vi "optimize crop parameters-3 (SubVI).vi"(6 "ref image in":u16[][](array[numeric])=array300x57[17100 elements], 7 "fit results":bool=TRUE, 8 "init values":dbl[][][](array[numeric]), 9 "use external int values":bool, 10 "config in":T4={"xy cut pos correct"=[[0.0], [0.0], [0.0], [0.0], [0.0], [0.0], [0.0], [0.0], [0.0], [0.0], [0.0], [0.0], [0.0], [0.0], [0.0], [0.0], [0.0], [0.0], [0.0], [0.0], [0.0], [0.0], [0.0], [0.0], [0.0], [0.0], [0.0], [0.0], [0.0], [0.0], [0.0], [0.0], [0.0], [0.0], [0.0], [0.0], [0.0], [0.0], [0.0], [0.0]], "3D reconst config"={"xyz pos"=[0, 69, 24], "color 4"={"color array"=[0, 8388736, 16711680, 16776960, 16776960, 16711680, 16448250, 16448250], "num of colors"=4, "max"=7000.900000000023, "min"=100.0}, "autogain"=TRUE, "zoom"=1.0, "slice(T)/stack(F)"=FALSE, "xy cut mag"=0.999999999999986, "xy cut ofst"=0.0, "z/xy comp"=0.9999999999999996, "y shift comp"=-7.0, "max plot"=TRUE, "oblique angle [deg]"=0.0, "voxel size z [um]"=0.36775838497734437, "voxel size xy[um]"=0.20475, "reverse v"=FALSE, "reverse h"=TRUE, "3D reconstruction"=TRUE, "reverse z"=FALSE}, "xy cut pos"=[[0.0], [54.34536278984456], [110.7007419058657], [167.1825518682615], [222.80744164966734], [279.667373495206], [337.55045867160084], [394.00066092240456], [449.7285684304855], [506.4608987736647], [563.3091240593538], [619.1119535504733], [675.221494909653], [732.8446944573865], [789.812326653542], [845.898454893022], [902.613225396426], [960.3441252947761], [1016.341283679399], [1071.7472607916166], [1127.5653088105405], [1184.377243760696], [1240.3662075534241], [1296.3844377457767], [1353.119109400925], [1408.8200918213527], [1464.8184208619614], [1521.6959125472738], [1579.4607614691888], [1635.079797970669], [1691.0593965155172], [1748.3068154920788], [1805.199525705196], [1861.439009878706], [1917.7054191398715], [1974.9902991079516], [2031.335142320107], [2087.3943454719315], [2144.892284829274], [2201.6960251875375]], "AOD scan speed ratio"=10.0, "Nx"=56.85, "stack method"=enum."0pad to x", "y shift"=-3}, 11 "image in":u16[][][](array[numeric])=array1x300x2304[691200 elements]) -> (0 "opt param for feedback":dbl[][][](array[numeric])=[[[0.39047108985224355, 1.3701514145414102, -2.528506798772906, -0.14203827683511228, 5186038.086192495]], [[0.5290682113405143, 1.6501694868561811, -2.655816972530653, -0.1554672078248204, 6667073.766870199]], [[0.41314522689268984, 2.088686528657111, -2.792705091791418, -0.12569963497559422, 6491844.329115606]], [[0.8227560588149236, 1.8428855088240716, -2.628942466676763, -0.08668976787454216, 5631903.835843649]], [[0.32325175994989747, 1.2513074134525095, -1.6297905856914976, -0.1614369028609812, 7505225.271223895]], [[-0.003655911531680436, 0.19950104929288875, -1.7514530723749357, -0.08884972633189654, 5034310.712258729]], [[0.34354411314901734, 1.2590913467770888, -2.7890670826012935, -0.10927959716588379, 6468144.578476399]], [[-0.0310203421500183, 0.7829252064146169, -2.2702759490200592, -0.09899784044930304, 4653169.175374532]], [[0.14511870715681918, 0.24470450605468053, -1.7093878850525326, -0.06709896777407671, 5134381.833655705]], [[-0.003971505084047196, 0.7523626416256568, -1.534678939554147, -0.09611567176314631, 4740038.50089103]], [[-0.02792801163393208, -0.3890095646502043, -2.2976472939935375, -0.09700731789796588, 5338166.755682839]], [[-0.6560035416703861, -0.4121475704316506, -1.8006560477706657, -0.08317774197600952, 4965586.880682849]], [[-0.07899279410231272, 0.5752260971778136, -0.6710344360087989, -0.06849372931756358, 4655084.0858172625]], [[-0.05083354360854886, 0.2532900218711269, -1.39597945278722, -0.07627262365560383, 5236824.424857916]], [[-0.04837211414479735, 0.3406051408186316, -0.7975973572536321, -0.08658047534428787, 4753028.594224306]], [[-0.4313850295473879, -0.6276284625697358, -0.7897096438499904, -0.072834398097467, 4874063.437715337]], [[-0.46049782115417903, -0.2341675376827123, -0.7412505694712552, -0.08633169971762658, 5141070.08632244]], [[0.08833028483609733, 0.8215796169595931, -0.01775522596758547, -0.06738233458537551, 4677016.607236656]], [[-0.6223872033178044, -0.9987743136212477, -1.0676478560072118, -0.03407086417350795, 5553505.071871417]], [[-0.017060112368393276, 1.0784317210282457, -0.2722875991586168, -0.0816359092925706, 4696857.4358025845]], [[0.0, 0.0, 0.0, 0.0, 0.0]], [[-0.23613314760922, 0.3409617993905103, 0.3289119936344964, -0.09632032650540112, 5128288.939512947]], [[-0.35196031039538767, 0.10630624968944505, 0.8300543336834989, -0.08524955580697285, 4993967.3927470865]], [[-0.029822860931065412, 0.5761693339828244, 0.009485866537335071, -0.072483002212926, 4951118.4930408215]], [[0.3466422521632596, 1.1972939848079962, 0.8529442246259615, -0.08204563144140758, 4738224.722203573]], [[-0.5161452276940326, -0.4062966847061925, 1.4794783929753714, -0.04368130498426906, 4589002.30593094]], [[-0.38498865045824193, 0.7296022962419677, 1.219223749125252, -0.08128900584448218, 5155405.171288024]], [[0.39664586657630685, 0.19347099987965855, 1.9179908940418189, -0.08728195443943998, 5146203.651410466]], [[-0.06294995676019306, 0.5468584220156103, 1.258683657908979, -0.07957290144422699, 4724989.578754336]], [[-0.5068124364570108, -0.08803959075677643, 2.2015231672130584, -0.07409643531910859, 4765076.553921852]], [[-0.007101178214248816, 0.10218423404460837, 2.4109047574004157, -0.06616032890532567, 4331638.820783317]], [[-0.41299002227983295, 1.1421701438972842, 1.8680971965858637, -0.10395219837168257, 5779592.647707423]], [[-0.04906443565345491, 0.2939222046041641, 1.9091893754914997, -0.04341744032696582, 4796031.169651782]], [[-0.06496644337617823, 0.5511641655160622, 1.91046003816149, -0.05321838499215621, 4379387.893441995]], [[-0.3555959703865873, 0.1452031874907217, 3.037388781526421, -0.052724460570182485, 4931796.160483034]], [[-0.4774462977628986, -0.44051726867204, 2.350105869256047, -0.0908046301186699, 5146929.721792191]], [[-0.45397018791592364, 0.3915383175697266, 3.3398737812628516, -0.07691847566668765, 4864469.550526747]], [[0.14328180351502526, 0.3855249139291015, 2.6047417917604205, -0.06972164986512942, 4334268.987205673]], [[-0.07403056676163042, 0.8482394818552436, 3.2115811981035, -0.09535149758334224, 4409611.6475773165]], [[-0.26001393141243034, 0.5649152359263228, 4.100365157728029, -0.09799498059142073, 5159717.129331669]]], 3 "optimized parameters":dbl[][][](array[numeric])=[[[0.6536916642864307, 9.691050019608873, -3.146642560188741, -0.1502911301649359]], [[0.5397363402674268, 65.0684934356392, -2.979252154665359, -0.13747551755601403]], [[0.4364891379835099, 120.61174935417779, -2.8118617491419773, -0.12770796069082646]], [[0.3433633747841549, 176.2986144777129, -2.644471343618595, -0.12005961729517042]], [[0.259784258948234, 232.1081618516672, -2.477080938095213, -0.11381811925822599]], [[0.18518888968401584, 288.0207408643976, -2.309690532571831, -0.10845694075667886]], [[0.11902625712916581, 344.01797724719563, -2.142300127048449, -0.1036067632845281]], [[0.06075724235074598, 400.08277307428693, -1.974909721525067, -0.0990288375885783]], [[0.009854617345215477, 456.19930676283155, -1.8075193160016851, -0.09459034250961632]], [[-0.03419695496157027, 512.353033072924, -1.6401289104783032, -0.09024174072927313]], [[-0.071900920714359, 568.5306831075931, -1.472738504954921, -0.0859961314225699]], [[-0.10374883512850164, 624.720264312802, -1.3053480994315392, -0.08191059981614907]], [[-0.1302203624899524, 680.9110604774485, -1.1379576939081573, -0.07806956365218976]], [[-0.15178327615526876, 737.0936317333643, -0.9705672883847751, -0.07457011655800833]], [[-0.16889345855161175, 793.2598145553159, -0.803176882861393, -0.07150936832134314]], [[-0.1819949011767451, 849.4027217610037, -0.6357864773380113, -0.06897378207132454]], [[-0.19151970459903644, 905.5167425110632, -0.46839607181462917, -0.06703050836512858]], [[-0.19788807845745615, 961.5975423090633, -0.30100566629124703, -0.06572071618031705]], [[-0.20150834146157814, 1017.6420630015082, -0.13361526076786534, -0.0650549208128599]], [[-0.20277692139158043, 1073.6485227778358, 0.033775144755516795, -0.06501030868084456]], [[-0.20207835509824212, 1129.6164161704187, 0.20116555027889893, -0.06553005903386944]], [[-0.1997852885029483, 1185.5465140545639, 0.3685559558022806, -0.06652466256812017]], [[-0.19625847659768425, 1241.440863648512, 0.5359463613256628, -0.06787523694713249]], [[-0.1918467834450428, 1297.3027885134397, 0.7033367668490449, -0.06943883922824079]], [[-0.1868871821782152, 1353.1368885534564, 0.8707271723724266, -0.07105577519470918]], [[-0.18170475500099958, 1408.9490400156064, 1.0381175778958087, -0.07255890559354494]], [[-0.17661269318779516, 1464.7463954898685, 1.2055079834191909, -0.07378494927900459]], [[-0.1719122970836069, 1520.537383909156, 1.372898388942573, -0.07458778326177828]], [[-0.16789297610403953, 1576.3317105493163, 1.5402887944659551, -0.07485373966385556]], [[-0.1648322487353049, 1632.1403570291309, 1.7076791999893364, -0.07451889957908975]], [[-0.16299574253421412, 1687.9755813103163, 1.8750696055127185, -0.07358838383942778]], [[-0.16263719412818567, 1743.850917697523, 2.0424600110361006, -0.07215764068684027]], [[-0.1639984492152391, 1799.781176838336, 2.2098504165594828, -0.07043573035093509]], [[-0.16730946256399637, 1855.7824457232746, 2.377240822082865, -0.06877060653223754]], [[-0.172788298013685, 1911.8720876857924, 2.544631227606247, -0.06767639479118515]], [[-0.18064112847413405, 1968.0687424022772, 2.712021633129629, -0.06786266784277828]], [[-0.1910622359257763, 2024.392325892052, 2.8794120386530104, -0.07026571775693569]], [[-0.2042340114196488, 2080.864030517373, 3.0468024441763926, -0.07608182506452543]], [[-0.22032695507739053, 2137.506324983432, 3.2141928496997747, -0.08680252476907313]], [[-0.23949967609124334, 2194.342954338354, 3.381583255223157, -0.10425186926418739]]])   [LabVIEW 2024]
uses:
  <vilib>/Analysis/6fits.llb/General Linear Fit Algorithm.ctl
  <vilib>/Analysis/6fits.llb/Curve Fitting Criteria.ctl
  <vilib>/Analysis/1siggen.llb/Ramp Pattern by Samples.vi
  Global variables/global for picoscope.vi
  <vilib>/gmath/NumericalOptimization/Conjugate Gradient.vi
  <vilib>/gmath/NumericalOptimization/Downhill Simplex.vi
  <vilib>/gmath/NI_Gmath.lvlib
  <vilib>/Analysis/NI_AALBase.lvlib
  <vilib>/Analysis/NI_AALPro.lvlib
panel:
  out "y correct":dbl[](array[numeric])
  out "intensity correct fit":dbl[][](graph)=[[-0.008252853329823617, 0.01799169026880637, -0.00200832571523224, -0.03336984942062826, 0.047618783602755205, -0.019607214424782318, 0.005672833881355685, -3.099713927526282e-05, -0.0274913747355396, 0.005873931033873181, 0.011011186475395979, 0.001267142159860457, -0.00957583433462618, 0.001702507097595507, 0.01507110702294473, 0.0038606160261424605, 0.019301191352498, 0.0016616184050584626, -0.030984056639351956, 0.016625600611726035, -0.06553005903386944, 0.029795663937280947, 0.017374318859840365, 0.0030441629846852114, 0.010989856246698404, -0.028877600609275883, 0.00750405656547759, 0.012694171177661695, 0.004719161780371434, -0.000422464259981159, -0.0074280549341021185, 0.031794557684842295, -0.02701829002396927, -0.015552221540081332, -0.01495193422100266, 0.022941962275891625, 0.0066527579097519635, -0.006360175199396009, 0.008548972814269112, -0.006256888672766664]]
  out "y correct fit":dbl[][](graph)=[[-0.6181357614158349, -0.3234351821347059, -0.01915665735055949, -0.015528876941832248, -0.8472903524037154, -0.5582374601968951, 0.6467669555528444, 0.2953662274949922, -0.09813143094915255, -0.10544997092415631, 0.8249087890386164, 0.4953079483391265, -0.4669232578993584, 0.4254121644024449, -0.005579525607760871, 0.15392316651197913, 0.27285449765662606, -0.28325044032366153, 0.9340325952393465, 0.3060627439141336, 0.20116555027889893, 0.03964396216778421, -0.29410797235783614, 0.6938509003117098, 0.01778294774646505, -0.4413608150795627, -0.013715765706061145, -0.5450925050992459, 0.28160513655697605, -0.49384396722372204, -0.5358351518876971, 0.17436281445023694, 0.3006610410679831, 0.4667807839213749, -0.49275755392017384, 0.3619157638735824, -0.4604617426098412, 0.44206065241597203, 0.0026116515962746334, -0.7187819025048721]]
  out "r correct fit":dbl[][](graph)=[[0.2632205744341871, 0.01066812892691249, 0.02334391109082007, -0.47939268403076873, -0.06346750100166348, 0.18884480121569627, -0.22451785601985152, 0.09177758450076427, -0.1352640898116037, -0.030225449877523073, -0.04397290908042692, 0.5522547065418845, -0.05122756838763967, -0.1009497325467199, -0.1205213444068144, 0.24939012837064278, 0.2689781165551426, -0.2862183632935535, 0.42087886185622625, -0.18571680902318716, -0.20207835509824212, 0.036347859106271696, 0.15570183379770342, -0.1620239225139774, -0.5335294343414748, 0.334440472693033, 0.20837595727044678, -0.5685581636599137, -0.10494301934384646, 0.3419801877217059, -0.1558945643199653, 0.2503528281516473, -0.11493401356178418, -0.10234301918781814, 0.1828076723729023, 0.29680516928876455, 0.2629079519901473, -0.3475158149346741, -0.1462963883157601, 0.020514255321187003]]
  out "x cut pos fit":dbl[][](graph)=[[0.05958342353034496, 0.3696472414168426, -0.5619591246160951, -0.507951857113909, -0.017269990121718592, 1.1759828176153064, -0.5767823185710199, -0.6787897339829101, 0.46230636415401705, -0.4421715948110432, 0.704871654653175, 1.0956096058057483, 0.08464138025601642, 0.2628733892471473, -0.6385644162365907, 0.6061678936717954, -0.22042479817071126, -1.4538074471773825, -0.10131294393795542, -1.3327500488101123, 0.5811761866887082, -0.25952303329358983, 0.5225790325855542, 0.27997021796568333, -1.2632396330939173, 1.5644171407125214, 0.3021165107622892, -0.17226765343639272, 0.22220656651415993, 0.9923966661572194, 0.7340449659257047, -0.6067568190055681, -0.3854211309949278, -0.34487591421111574, -0.3506291171152043, 0.27174445488094534, -0.9228543205397273, -0.358506167194264, 0.28250261545827016, 0.6210199346419358]]
  out "x cut correct 3":dbl[](graph)=[1.3701514145414102, 1.6501694868561811, 2.088686528657111, 1.8428855088240716, 1.2513074134525095, 0.19950104929288875, 1.2590913467770888, 0.7829252064146169, 0.24470450605468053, 0.7523626416256568, -0.3890095646502043, -0.4121475704316506, 0.5752260971778136, 0.2532900218711269, 0.3406051408186316, -0.6276284625697358, -0.2341675376827123, 0.8215796169595931, -0.9987743136212477, 1.0784317210282457, 0.0, 0.3409617993905103, 0.10630624968944505, 0.5761693339828244, 1.1972939848079962, -0.4062966847061925, 0.7296022962419677, 0.19347099987965855, 0.5468584220156103, -0.08803959075677643, 0.10218423404460837, 1.1421701438972842, 0.2939222046041641, 0.5511641655160622, 0.1452031874907217, -0.44051726867204, 0.3915383175697266, 0.3855249139291015, 0.8482394818552436, 0.5649152359263228]
  out "x cut correct 2":dbl[](graph)=[-0.8029671311863609, -1.22048533842898, -0.20099096700753716, -2.396117725234003, -0.5704273524019985, 0.2214525690458135, -0.6696516702608777, 0.9702091819145723, -0.6014491907781662, 0.7762106145991239, -0.22050026893236452, 4.118267322604225, 1.0567908915209814, 0.5614239918423856, 0.6336730889351082, 2.205079255222368, 2.8091033079627183, 0.30079806451595614, 3.266476398749979, 1.1811428479118296, 0.0, 1.827987916571229, 2.3779756021428033, 0.756180187298116, -0.7477150646922253, 3.0470615566129515, 3.2322309224736365, -2.0114867259898572, 0.9293740307831726, 3.295832744570641, 0.1448519014721809, 3.843210849841621, 0.5912262293633566, 0.9460942665828354, 2.4421349452744177, 2.7265847440253017, 3.387362410336551, -0.45021659697024496, 1.2990983499316635, 2.2105778664701514]
  out "size(s)":i32[](array[numeric])=[40, 1]
  out "loss function":dbl[](graph)=[5186038.086192495, 6667073.766870199, 6491844.329115606, 5631903.835843649, 7505225.271223895, 5034310.712258729, 6468144.578476399, 4653169.175374532, 5134381.833655705, 4740038.50089103, 5338166.755682839, 4965586.880682849, 4655084.0858172625, 5236824.424857916, 4753028.594224306, 4874063.437715337, 5141070.08632244, 4677016.607236656, 5553505.071871417, 4696857.4358025845, 0.0, 5128288.939512947, 4993967.3927470865, 4951118.4930408215, 4738224.722203573, 4589002.30593094, 5155405.171288024, 5146203.651410466, 4724989.578754336, 4765076.553921852, 4331638.820783317, 5779592.647707423, 4796031.169651782, 4379387.893441995, 4931796.160483034, 5146929.721792191, 4864469.550526747, 4334268.987205673, 4409611.6475773165, 5159717.129331669]
  out "intensity correct":dbl[][](graph)=[[-0.14203827683511228, -0.1554672078248204, -0.12569963497559422, -0.08668976787454216, -0.1614369028609812, -0.08884972633189654, -0.10927959716588379, -0.09899784044930304, -0.06709896777407671, -0.09611567176314631, -0.09700731789796588, -0.08317774197600952, -0.06849372931756358, -0.07627262365560383, -0.08658047534428787, -0.072834398097467, -0.08633169971762658, -0.06738233458537551, -0.03407086417350795, -0.0816359092925706, 0.0, -0.09632032650540112, -0.08524955580697285, -0.072483002212926, -0.08204563144140758, -0.04368130498426906, -0.08128900584448218, -0.08728195443943998, -0.07957290144422699, -0.07409643531910859, -0.06616032890532567, -0.10395219837168257, -0.04341744032696582, -0.05321838499215621, -0.052724460570182485, -0.0908046301186699, -0.07691847566668765, -0.06972164986512942, -0.09535149758334224, -0.09799498059142073], [-0.1502911301649359, -0.13747551755601403, -0.12770796069082646, -0.12005961729517042, -0.11381811925822599, -0.10845694075667886, -0.1036067632845281, -0.0990288375885783, -0.09459034250961632, -0.09024174072927313, -0.0859961314225699, -0.08191059981614907, -0.07806956365218976, -0.07457011655800833, -0.07150936832134314, -0.06897378207132454, -0.06703050836512858, -0.06572071618031705, -0.0650549208128599, -0.06501030868084456, -0.06553005903386944, -0.06652466256812017, -0.06787523694713249, -0.06943883922824079, -0.07105577519470918, -0.07255890559354494, -0.07378494927900459, -0.07458778326177828, -0.07485373966385556, -0.07451889957908975, -0.07358838383942778, -0.07215764068684027, -0.07043573035093509, -0.06877060653223754, -0.06767639479118515, -0.06786266784277828, -0.07026571775693569, -0.07608182506452543, -0.08680252476907313, -0.10425186926418739]]
  out "y correct":dbl[][](graph)=[[-2.528506798772906, -2.655816972530653, -2.792705091791418, -2.628942466676763, -1.6297905856914976, -1.7514530723749357, -2.7890670826012935, -2.2702759490200592, -1.7093878850525326, -1.534678939554147, -2.2976472939935375, -1.8006560477706657, -0.6710344360087989, -1.39597945278722, -0.7975973572536321, -0.7897096438499904, -0.7412505694712552, -0.01775522596758547, -1.0676478560072118, -0.2722875991586168, 0.0, 0.3289119936344964, 0.8300543336834989, 0.009485866537335071, 0.8529442246259615, 1.4794783929753714, 1.219223749125252, 1.9179908940418189, 1.258683657908979, 2.2015231672130584, 2.4109047574004157, 1.8680971965858637, 1.9091893754914997, 1.91046003816149, 3.037388781526421, 2.350105869256047, 3.3398737812628516, 2.6047417917604205, 3.2115811981035, 4.100365157728029], [-3.146642560188741, -2.979252154665359, -2.8118617491419773, -2.644471343618595, -2.477080938095213, -2.309690532571831, -2.142300127048449, -1.974909721525067, -1.8075193160016851, -1.6401289104783032, -1.472738504954921, -1.3053480994315392, -1.1379576939081573, -0.9705672883847751, -0.803176882861393, -0.6357864773380113, -0.46839607181462917, -0.30100566629124703, -0.13361526076786534, 0.033775144755516795, 0.20116555027889893, 0.3685559558022806, 0.5359463613256628, 0.7033367668490449, 0.8707271723724266, 1.0381175778958087, 1.2055079834191909, 1.372898388942573, 1.5402887944659551, 1.7076791999893364, 1.8750696055127185, 2.0424600110361006, 2.2098504165594828, 2.377240822082865, 2.544631227606247, 2.712021633129629, 2.8794120386530104, 3.0468024441763926, 3.2141928496997747, 3.381583255223157]]
  out "x cut pos":dbl[][](graph)=[[9.631466596078528, 64.69884619422236, 121.17370847879388, 176.8065663348268, 232.12543184178892, 286.8447580467823, 344.59475956576665, 400.76156280826984, 455.73700039867754, 512.795204667735, 567.8258114529399, 623.6246547069962, 680.8264190971925, 736.8307583441172, 793.8983789715525, 848.7965538673319, 905.7371673092339, 963.0513497562407, 1017.7433759454461, 1074.9812728266459, 1129.03523998373, 1185.8060370878575, 1240.9182846159265, 1297.022818295474, 1354.4001281865503, 1407.384622874894, 1464.4442789791062, 1520.7096515625924, 1576.1095039828022, 1631.1479603629737, 1687.2415363443906, 1744.4576745165286, 1800.166597969331, 1856.1273216374857, 1912.2227168029076, 1967.7969979473962, 2025.3151802125917, 2081.2225366845673, 2137.2238223679738, 2193.721934403712], [9.691050019608873, 65.0684934356392, 120.61174935417779, 176.2986144777129, 232.1081618516672, 288.0207408643976, 344.01797724719563, 400.08277307428693, 456.19930676283155, 512.353033072924, 568.5306831075931, 624.720264312802, 680.9110604774485, 737.0936317333643, 793.2598145553159, 849.4027217610037, 905.5167425110632, 961.5975423090633, 1017.6420630015082, 1073.6485227778358, 1129.6164161704187, 1185.5465140545639, 1241.440863648512, 1297.3027885134397, 1353.1368885534564, 1408.9490400156064, 1464.7463954898685, 1520.537383909156, 1576.3317105493163, 1632.1403570291309, 1687.9755813103163, 1743.850917697523, 1799.781176838336, 1855.7824457232746, 1911.8720876857924, 1968.0687424022772, 2024.392325892052, 2080.864030517373, 2137.506324983432, 2194.342954338354]]
  out "r correct":dbl[][](graph)=[[0.39047108985224355, 0.5290682113405143, 0.41314522689268984, 0.8227560588149236, 0.32325175994989747, -0.003655911531680436, 0.34354411314901734, -0.0310203421500183, 0.14511870715681918, -0.003971505084047196, -0.02792801163393208, -0.6560035416703861, -0.07899279410231272, -0.05083354360854886, -0.04837211414479735, -0.4313850295473879, -0.46049782115417903, 0.08833028483609733, -0.6223872033178044, -0.017060112368393276, 0.0, -0.23613314760922, -0.35196031039538767, -0.029822860931065412, 0.3466422521632596, -0.5161452276940326, -0.38498865045824193, 0.39664586657630685, -0.06294995676019306, -0.5068124364570108, -0.007101178214248816, -0.41299002227983295, -0.04906443565345491, -0.06496644337617823, -0.3555959703865873, -0.4774462977628986, -0.45397018791592364, 0.14328180351502526, -0.07403056676163042, -0.26001393141243034], [0.6536916642864307, 0.5397363402674268, 0.4364891379835099, 0.3433633747841549, 0.259784258948234, 0.18518888968401584, 0.11902625712916581, 0.06075724235074598, 0.009854617345215477, -0.03419695496157027, -0.071900920714359, -0.10374883512850164, -0.1302203624899524, -0.15178327615526876, -0.16889345855161175, -0.1819949011767451, -0.19151970459903644, -0.19788807845745615, -0.20150834146157814, -0.20277692139158043, -0.20207835509824212, -0.1997852885029483, -0.19625847659768425, -0.1918467834450428, -0.1868871821782152, -0.18170475500099958, -0.17661269318779516, -0.1719122970836069, -0.16789297610403953, -0.1648322487353049, -0.16299574253421412, -0.16263719412818567, -0.1639984492152391, -0.16730946256399637, -0.172788298013685, -0.18064112847413405, -0.1910622359257763, -0.2042340114196488, -0.22032695507739053, -0.23949967609124334]]
  out "slice":i32=39
  out "page":i32
  out "Numeric":i32=9
  out "Waveform Graph 3":dbl[](graph)=[0.0, 0.0, 7.072244388269059e-25, 0.0, 0.0, 1251222.7679371487, 0.0, 0.0, 0.0, 1886418.1063101203]
  out "x-y":dbl=6.488273299997672
  out "sum 2":dbl
  out "difference from ref img":dbl[][](graph)
  out "error out":errorcluster
  in  "Conjugate gradient settings":T1
  in  "Stopping criteria":T2={"function tolerance"=1000.0, "parameter tolerance"=0.1, "max iterations"=1000, "max function calls"=1000, "gradient tolerance"=-1.0, "max time (sec)"=-1.0}
  in  "Optimization Method":T3(ring)=enum."Downhill Simplex"
  out "Number of function evaluations":i32=89
  out "Minimum":dbl[](array[numeric])
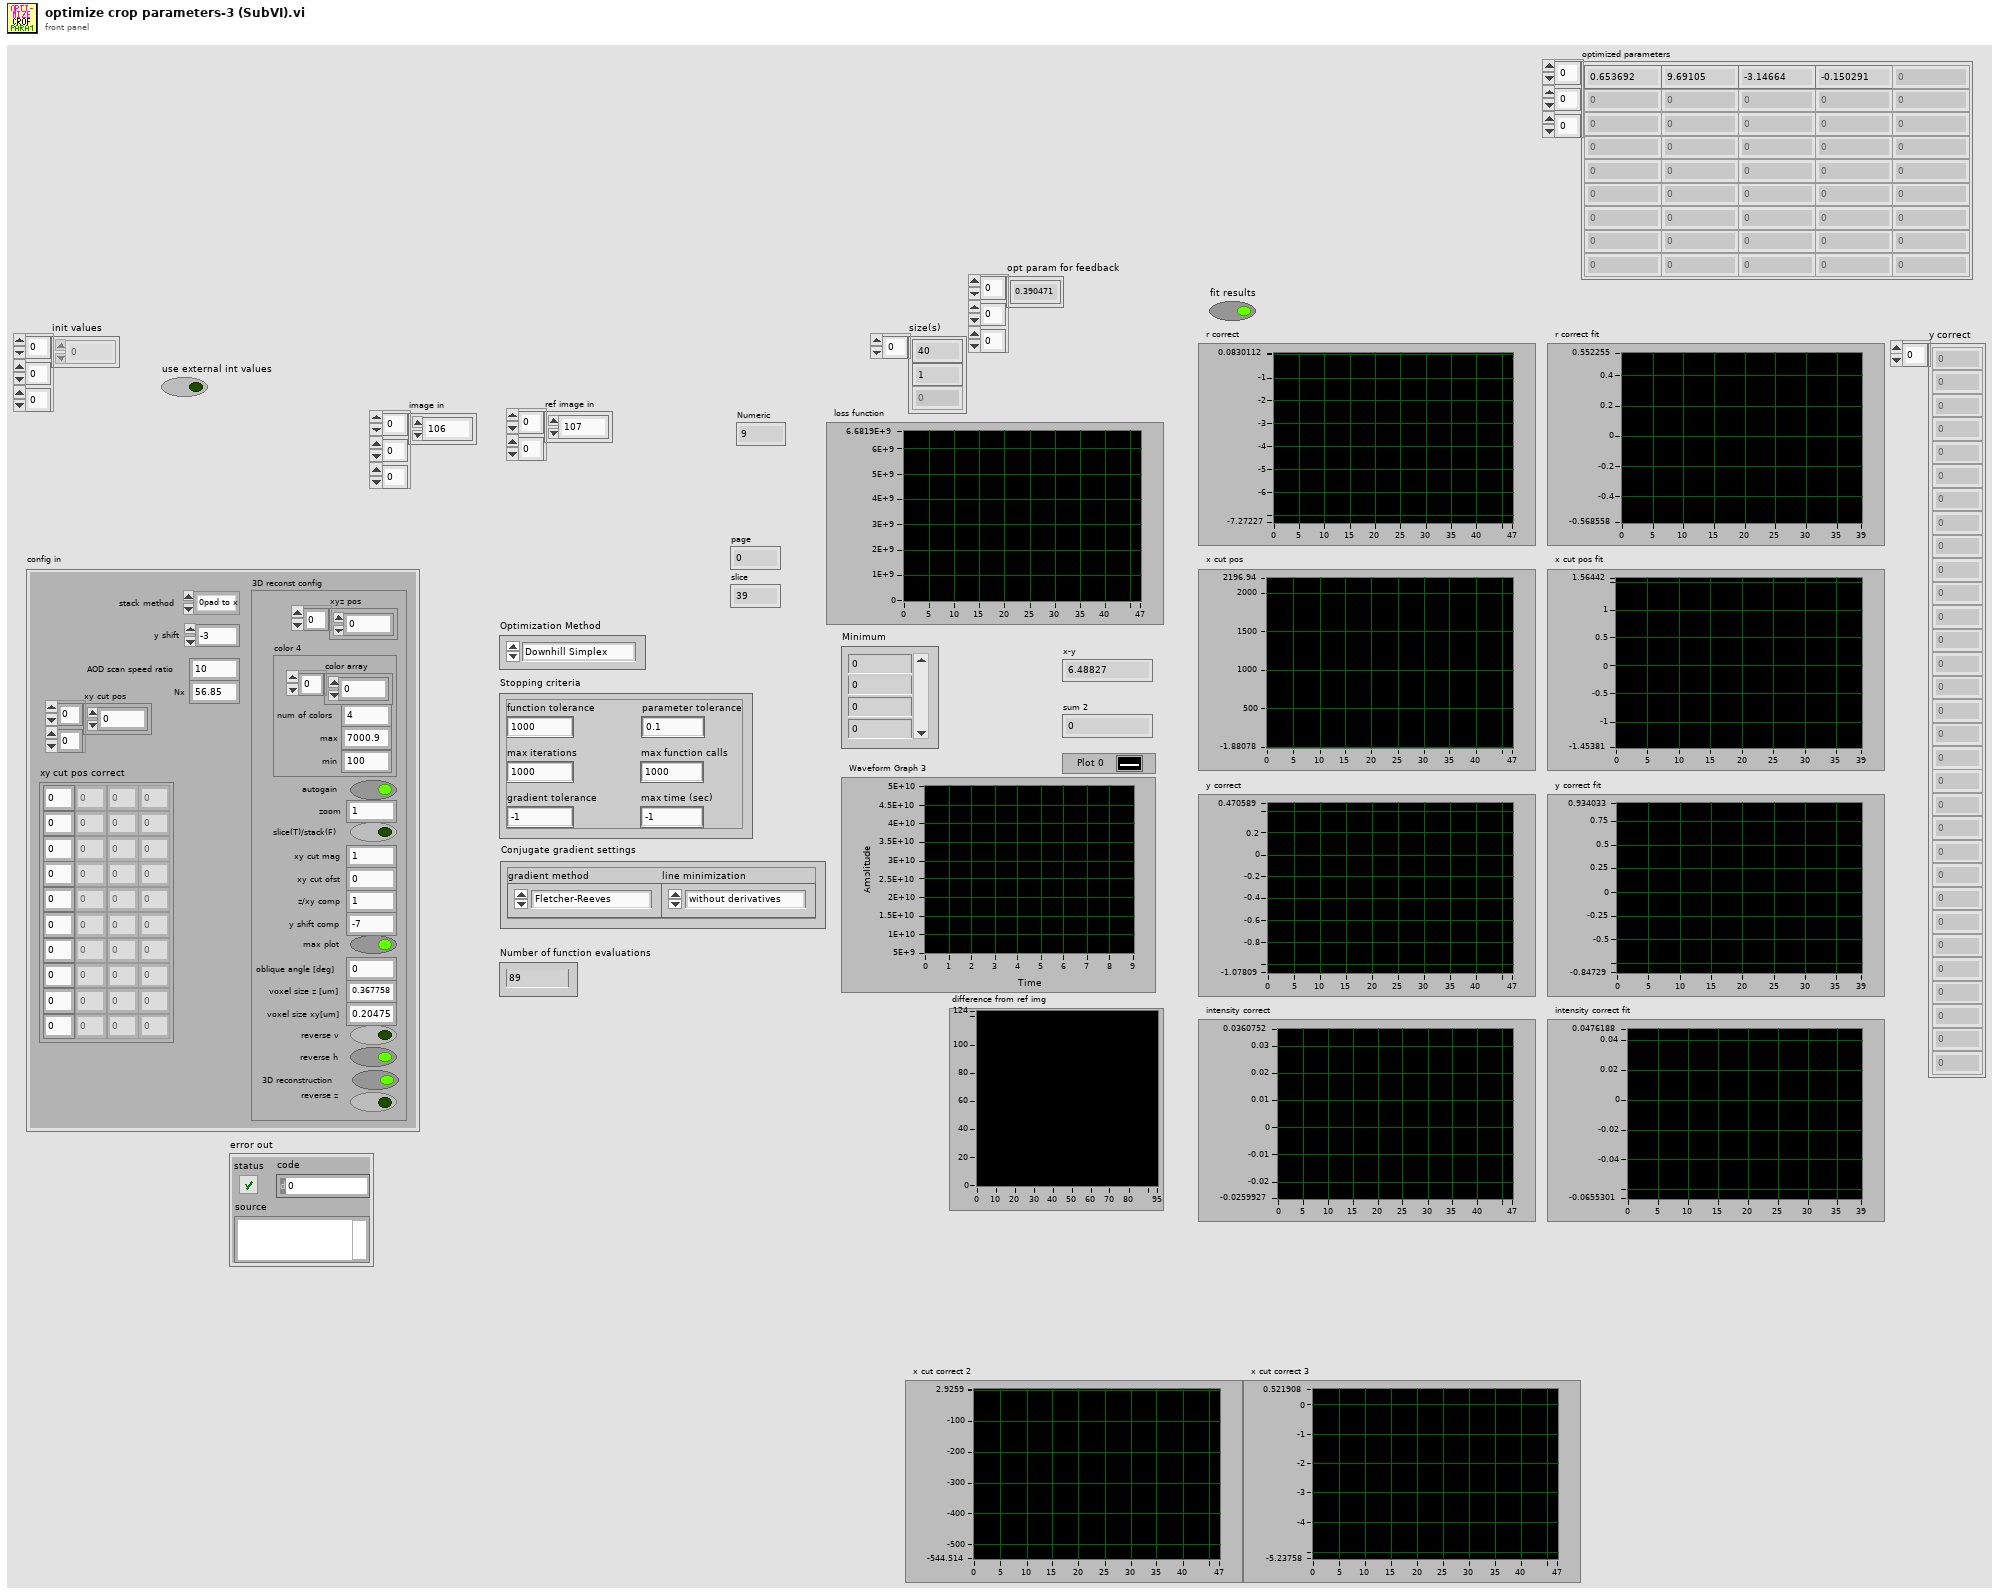
[diagram p1: front panel]
types:
  T1 = cluster{"gradient method":enum16{"Fletcher-Reeves", "Polak-Ribiere"}, "line minimization":enum16{"without derivatives", "with derivatives"}}
  T2 = cluster{"function tolerance":dbl, "parameter tolerance":dbl, "max iterations":i32, "max function calls":i32, "gradient tolerance":dbl, "max time (sec)":dbl}
  T3 = enum16{"Quasi-newton", "Conjugate Gradient", "Downhill Simplex"}
  T4 = cluster{"xy cut pos correct":dbl[][], "3D reconst config":cluster{"xyz pos":u16[], "color 4":cluster{"color array":u32[], "num of colors":i32, "max":dbl, "min":dbl}, "autogain":bool, "zoom":dbl, "slice(T)/stack(F)":bool, "xy cut mag":dbl, "xy cut ofst":dbl, "z/xy comp":dbl, "y shift comp":dbl, "max plot":bool, "oblique angle [deg]":dbl, "voxel size z [um]":dbl, "voxel size xy[um]":dbl, "reverse v":bool, "reverse h":bool, "3D reconstruction":bool, "reverse z":bool}, "xy cut pos":dbl[][], "AOD scan speed ratio":dbl, "Nx":dbl, "stack method":enum16{"0pad to z", "0pad to x", "0pad to x and rot"}, "y shift":i32}
  T5 = cluster{"xyz pos":u16[], "color 4":cluster{"color array":u32[], "num of colors":i32, "max":dbl, "min":dbl}, "autogain":bool, "zoom":dbl, "slice(T)/stack(F)":bool, "xy cut mag":dbl, "xy cut ofst":dbl, "z/xy comp":dbl, "y shift comp":dbl, "max plot":bool, "oblique angle [deg]":dbl, "voxel size z [um]":dbl, "voxel size xy[um]":dbl, "reverse v":bool, "reverse h":bool, "3D reconstruction":bool, "reverse z":bool}
  T6 = cluster{"GT":dbl[][], "frame input":u16[][], "cut pos init":dbl, "Nx":dbl, "r init":dbl}
  T7 = typedef "NI_AALPro.lvlib/General Linear Fit Algorithm.ctl" = u16
  T8 = typedef "NI_AALPro.lvlib/Curve Fitting Criteria.ctl" = u16
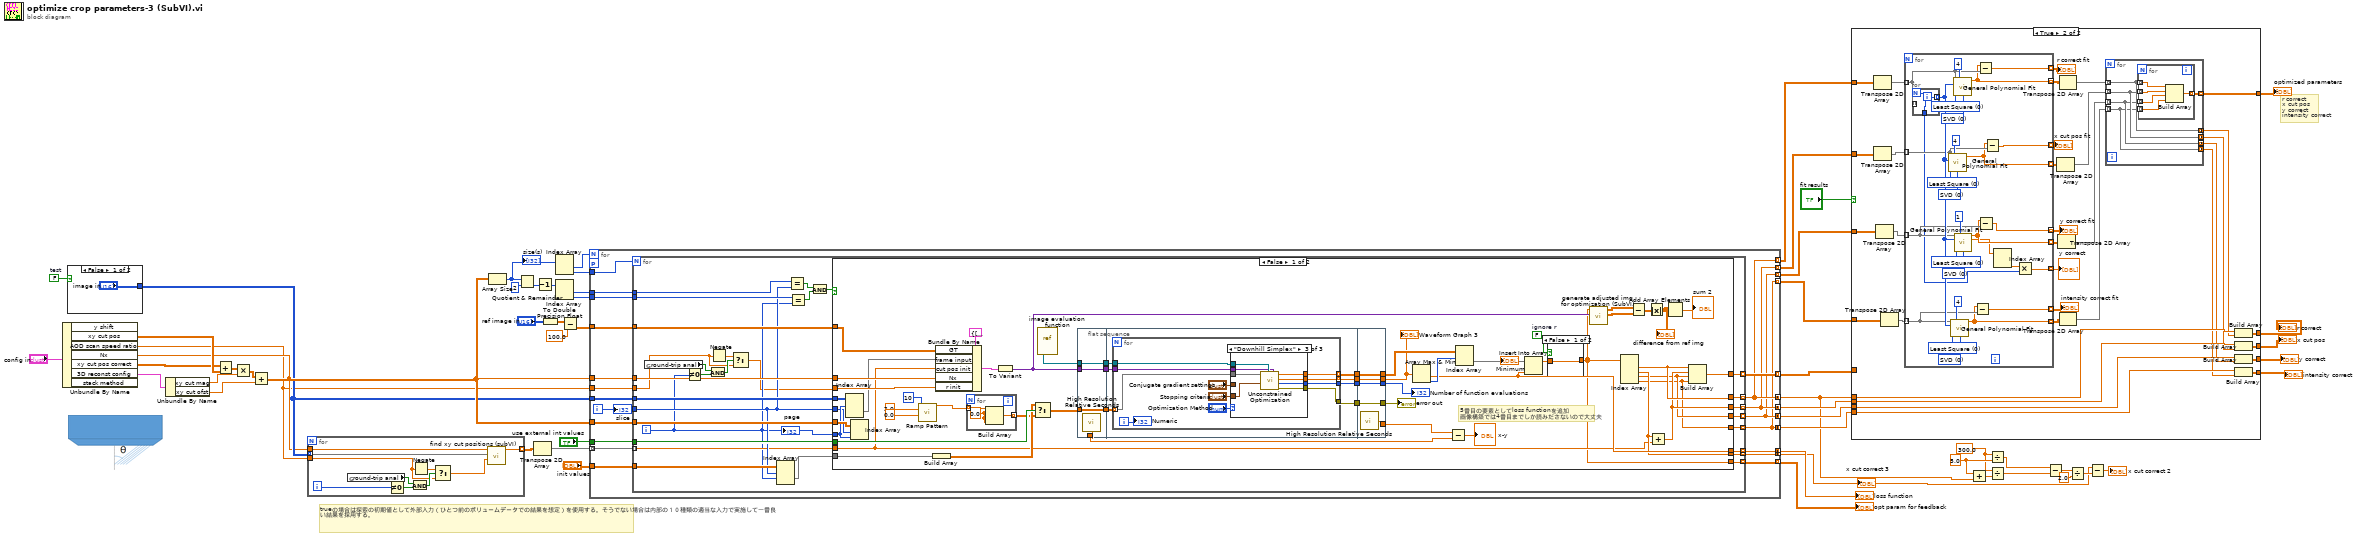
[diagram p0: block diagram]
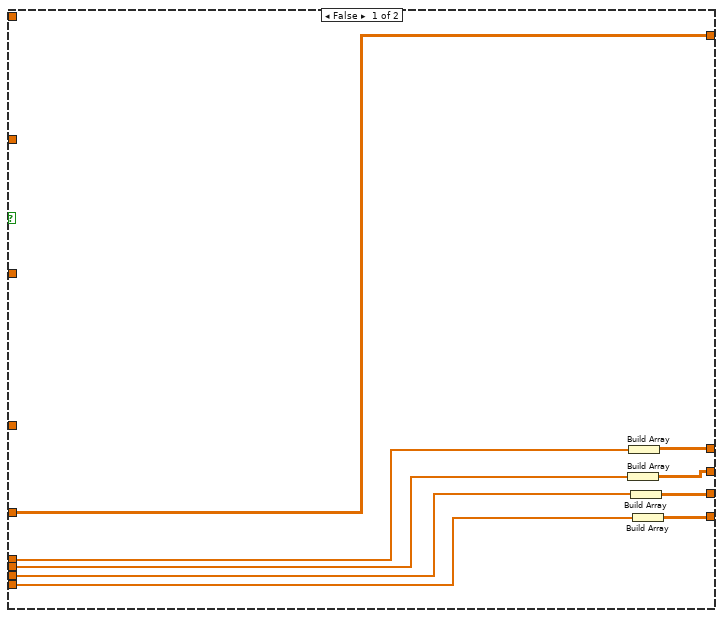
[diagram p2: hidden frame]
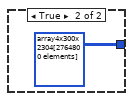
[diagram p3: hidden frame]
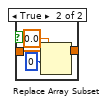
[diagram p4: hidden frame]
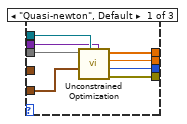
[diagram p5: hidden frame]
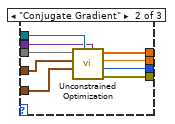
[diagram p6: hidden frame]
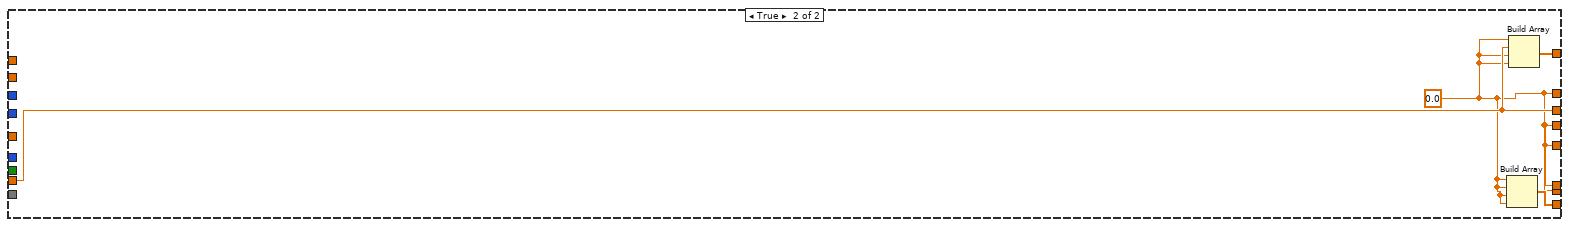
[diagram p7: hidden frame]
diagram:
  w28 = 5.0 ("y")
  w27 = 300.0 ("x")
  w37 = FALSE  # test
  # "r correct\nx cut pos\ny correct\nintensity correct"
  # "trueの場合は探索の初期値として外部入力（ひとつ前のボリュームデータでの結果を想定）を使用する。そうでない場合は内部の１０種類の適当な入力で実施して一番良い結果を採用する。"
  n1 = Unbundle By Name("config in") -> ("xy cut pos"=w55:dbl[][], "AOD scan speed ratio"=w33:dbl, "Nx"=w34:dbl, "xy cut pos correct"=w54:dbl[][], "3D reconst config"=w53:T5)  [unwired: 2 out]
  n2 = case shown="False" w37 {
    tunnel: ["image in" u16[][][] array4x300x2304[2764800 elements] ("Array out")] -> w35
    frame False {
    }
    frame True {
    }
  }
  n3 = Unbundle By Name(w53) -> ("xy cut mag"=w51:dbl, "xy cut ofst"=w49:dbl)
  n4 = Add(x=w54, y=w55) -> (x+y=w52:dbl[][])
  n5 = Multiply(x=w52, y=w51) -> (x*y=w50:dbl[][])
  n6 = Add(x=w50, y=w49) -> (x+y=w45:dbl[][])
  n7 = for {
    tunnel: w35 -> [w68] mode=indexing
    tunnel: w34 -> [w61]
    tunnel: w33 -> [w60]
    tunnel: [w67] -> w32 mode=indexing
    i -> [w63]
    n8 = global read "global for picoscope.vi" "round-trip anal"() -> (w64:bool)
    n9 = Not Equal To 0?(x=w63) -> (x != 0?=w62:bool)
    n10 = And(x=w64, y=w62) -> (x .and. y?=w65:bool)
    n11 = Negate(x=w60) -> (-x=w66:dbl)
    n12 = Select(t=w66, s=w65, f=w60) -> (s? t:f=w59:dbl)
    n13 = call "find xy cut positions (subVI).vi"("r"=w59, "input frame"=w68, "Nx"=w61) -> ("xy cut positions"=w67:dbl[])  [unwired: 7 in, 1 out]
  }
  n14 = Array Size(array=w45) -> (size(s)=w41:i32[])
  "size(s)" <- w41
  n15 = Quotient & Remainder(x=w41, y=2) -> (floor(x/y)=w43:i32[])  [unwired: 1 out]
  n16 = Transpose 2D Array(2D array=w32) -> (transposed array=w29:dbl[][])
  n17 = Decrement(x=w43) -> (x-1=w42:i32[])
  n18 = To Double Precision Float(number="ref image in") -> (double precision float=w48:dbl[][])
  n19 = Index Array(array=w41) -> (element #1=w17:i32, element #2=w16:i32)  [unwired: 2 in]
  n20 = Index Array(array=w42) -> (element #1=w39:i32, element #2=w38:i32)  [unwired: 2 in]
  n21 = Subtract(x=w48, y=100.0) -> (x-y=w46:dbl[][])
  n22 = for {
    N: w17 -> [_]
    tunnel: w35 -> [w88]
    tunnel: w34 -> [w87]
    tunnel: w33 -> [w86]
    tunnel: w46 -> [w85]
    tunnel: w45 -> [w84]
    tunnel: [w82] -> w10 mode=indexing
    tunnel: [w72] -> w1 mode=concatenating
    tunnel: [w81] -> w19 mode=concatenating
    tunnel: [w70] -> w7 mode=concatenating
    tunnel: [w69] -> w6 mode=concatenating
    tunnel: w16 -> [w78]
    tunnel: [w80] -> w40 mode=concatenating
    tunnel: w39 -> [w79]
    tunnel: w38 -> [w77]
    tunnel: "use external int values" -> [w76]
    tunnel: "init values" -> [w75]
    tunnel: w29 -> [w74] mode=indexing
    tunnel: [w71] -> w8 mode=concatenating
    tunnel: [w73] -> w18 mode=indexing
    tunnel: [w72] -> w15 mode=indexing
    tunnel: [w71] -> w14 mode=indexing
    tunnel: [w70] -> w13 mode=indexing
    tunnel: [w69] -> w12 mode=indexing
    workers-P: _ -> [_]
    i -> [w83]
    n23 = for {
      N: w78 -> [_]
      tunnel: w88 -> [w117]
      tunnel: w87 -> [w116]
      tunnel: w86 -> [w90]
      tunnel: w85 -> [w115]
      tunnel: w84 -> [w114]
      tunnel: w83 -> [w100]
      tunnel: [w113] -> w82 mode=indexing
      tunnel: [w112] -> w72 mode=indexing
      tunnel: [w111] -> w81 mode=indexing
      tunnel: [w110] -> w70 mode=indexing
      tunnel: [w109] -> w69 mode=indexing
      tunnel: [w108] -> w80 mode=indexing
      tunnel: w79 -> [w107]
      tunnel: w77 -> [w103]
      tunnel: w76 -> [w102]
      tunnel: w75 -> [w101]
      tunnel: w74 -> [w99] mode=indexing
      tunnel: [w98] -> w71 mode=indexing
      tunnel: [w97] -> w73 mode=indexing
      i -> [w92]
      n24 = global read "global for picoscope.vi" "round-trip anal"() -> (w95:bool)
      n25 = Not Equal To 0?(x=w92) -> (x != 0?=w94:bool)
      n26 = And(x=w95, y=w94) -> (x .and. y?=w93:bool)
      n27 = Negate(x=w90) -> (-x=w91:dbl)
      n28 = Select(t=w91, s=w93, f=w90) -> (s? t:f=w89:dbl)
      n29 = Index Array(array=w101, index (dim 0)=w100, index (dim 1)=w92) -> (element=w96:dbl[])  [unwired: 1 in]
      n30 = Equal?(x=w107, y=w100) -> (x = y?=w106:bool)
      n31 = Equal?(x=w103, y=w92) -> (x = y?=w105:bool)
      n32 = And(x=w106, y=w105) -> (x .and. y?=w104:bool)
      n33 = case shown="False" w104 {
        tunnel: w117 -> [w163 _]
        tunnel: w116 -> [w160 _]
        tunnel: w89 -> [w159 _]
        tunnel: w115 -> [w133 _]
        tunnel: w114 -> [w140 _]
        tunnel: w92 -> [w139 _]
        tunnel: w100 -> [w138 _]
        tunnel: [w123 w234] -> w113
        tunnel: [w127 w231] -> w112
        tunnel: [w129 w231] -> w111
        tunnel: [w125 w231] -> w110
        tunnel: [w124 w231] -> w109
        tunnel: [w134 w231] -> w108
        tunnel: w102 -> [w137 _]
        tunnel: w96 -> [w136 _]
        tunnel: w99 -> [w128 w233]
        tunnel: [w126 w233] -> w98
        tunnel: [w121 w232] -> w97
        frame False {
          w120 = FALSE  # ignore r
          # "5番目の要素としてloss functionを追加\n画像構築では4番目までしか読みださないので大丈夫"
          n34 = Index Array(array=w163, index (dim 0)=w139) -> (element=w141:u16[][])  [unwired: 2 in]
          n35 = Index Array(array=w140, index (row)=w138, index (col)=w139) -> ()  [unwired: 1 out]
          n36 = call-poly <vilib>:"Ramp Pattern.vi"("start"=0.0, "end"=2.0, "samples"=10) -> ("Ramp Pattern"=w148:dbl[])  [unwired: 7 in, 1 out]
          n37 = Build Array(w136) -> (w132:dbl[][])
          n38 = Bundle By Name(cluster=T6 {"GT"=[], "frame input"=[], "cut pos init"=0.0, "Nx"=0.0, "r init"=0.0}, "GT"=w133, "frame input"=w141, "cut pos init"=w128, "Nx"=w160, "r init"=w159) -> (w158:T6)
          n39 = for {
            tunnel: w148 -> [w230] mode=indexing
            tunnel: [w228] -> w131 mode=indexing
            w229 = 0.0 ("element")
            n40 = Build Array(w230, w229, w229, w229) -> (w228:dbl[])
          }
          n41 = To Variant(anything=w158) -> (Variant=w156:variant)
          n42 = Select(t=w132, s=w137, f=w131) -> (s? t:f=w130:dbl[][])
          n43 = vi-ref "image evaluation function.vi"() -> (w147:refnum<vi>)
          n44 = flat-sequence {
            tunnel: w147 -> [w177]
            tunnel: w130 -> [w178]
            tunnel: w156 -> [w179]
            tunnel: [w179] -> w170
            tunnel: [w178] -> w169
            tunnel: [w177] -> w168
            tunnel: [w176] -> w143
            tunnel: w170 -> [w184]
            tunnel: w169 -> [w183]
            tunnel: w168 -> [w182]
            tunnel: [w186] -> w167
            tunnel: [w185] -> w166
            tunnel: [w181] -> w165
            tunnel: [w180] -> w164
            tunnel: [w224] -> w145
            tunnel: [w225] -> w146
            tunnel: [w226] -> w157
            tunnel: [w227] -> w162
            tunnel: w167 -> [w227]
            tunnel: w166 -> [w226]
            tunnel: w165 -> [w225]
            tunnel: w164 -> [w224]
            tunnel: [w223] -> w142
            frame #0 {
              n45 = call <vilib>:"High Resolution Relative Seconds.vi"() -> ("relative seconds"=w176:dbl)
            }
            frame #1 {
              n46 = for {
                tunnel: [w197] -> w186
                tunnel: [w195] -> w180 mode=indexing
                tunnel: [w192] -> w185
                tunnel: w184 -> [w191]
                tunnel: [w190] -> w181 mode=indexing
                tunnel: w183 -> [w189] mode=indexing
                tunnel: w182 -> [w188]
                i -> [w187]
                n47 = case shown="\"Downhill Simplex\"" "Optimization Method" {
                  tunnel: w189 -> [w198 w206 w215]
                  tunnel: [w205 w214 w222] -> w197
                  tunnel: "Stopping criteria" -> [w204 w213 w221]
                  tunnel: [w203 w212 w220] -> w190
                  tunnel: [w202 w211 w219] -> w195
                  tunnel: [w201 w210 w218] -> w192
                  tunnel: "Conjugate gradient settings" -> [_ w209 _]
                  tunnel: w188 -> [w200 w208 w217]
                  tunnel: w191 -> [w199 w207 w216]
                  frame "Quasi-newton", Default {
                    n48 = call-poly <vilib>:"Unconstrained Optimization.vi"("function data"=w199, "objective function"=w200, "stopping criteria"=w204, "start"=w198) -> ("error out"=w201:errorcluster, "number of function evaluations"=w205:i32, "f(minimum)"=w202:dbl, "minimum"=w203:dbl[])  [unwired: 4 in]
                  }
                  frame "Conjugate Gradient" {
                    n49 = call-poly <vilib>:"Unconstrained Optimization.vi"("function data"=w207, "objective function"=w208, "stopping criteria"=w213, "conjugate gradient settings"=w209, "start"=w206) -> ("error out"=w210:errorcluster, "number of function evaluations"=w214:i32, "f(minimum)"=w211:dbl, "minimum"=w212:dbl[])  [unwired: 3 in]
                  }
                  frame "Downhill Simplex" {
                    n50 = call-poly <vilib>:"Unconstrained Optimization.vi"("function data"=w216, "objective function"=w217, "stopping criteria"=w221, "start"=w215) -> ("error out"=w218:errorcluster, "number of function evaluations"=w222:i32, "f(minimum)"=w219:dbl, "minimum"=w220:dbl[])  [unwired: 4 in]
                  }
                }
                "Numeric" <- w187
              }
            }
            frame #2 {
              n51 = call <vilib>:"High Resolution Relative Seconds.vi"() -> ("relative seconds"=w223:dbl)
            }
          }
          n52 = Array Max & Min(array=w145) -> (min value=w134:dbl, min index (indices)=w144:i32)  [unwired: 2 out]
          n53 = Subtract(x=w142, y=w143) -> (x-y=→"x-y":dbl)
          n54 = Index Array(array=w146, index (row)=w144) -> (element=w135:dbl[])  [unwired: 1 in]
          "Minimum" <- w135
          n55 = Insert Into Array(array=w135, new element=w134) -> (w122:dbl[])  [unwired: 1 in]
          n56 = case shown="False" w120 {
            tunnel: w122 -> [w171 w175]
            tunnel: [w171 w174] -> w121
            frame False {
            }
            frame True {
              n57 = Replace Array Subset(array=w175, new element=0.0 ("new element/subarray"), index=0) -> (w174:dbl[])
            }
          }
          n58 = call "generate adjusted img for optimization (SubVI).vi"("data"=w156, "X"=w121) -> ("Array"=w118:dbl[][], "GT"=w119:dbl[][])  [unwired: 7 in, 1 out]
          n59 = Index Array(array=w121) -> (element #1=w127:dbl, element #2=w129:dbl, element #3=w125:dbl, element #4=w124:dbl)  [unwired: 4 in]
          n60 = Subtract(x=w119, y=w118) -> (x-y=w155:dbl[][])
          n61 = Absolute Value(x=w155) -> (abs(x)=w154:dbl[][])
          "difference from ref img" <- w154
          n62 = Add(x=w129, y=w128) -> (x+y=w126:dbl)
          n63 = Add Array Elements(numeric array=w154) -> (sum=→"sum 2":dbl)
          n64 = Build Array(w127, w126, w125, w124) -> (w123:dbl[])
          "Number of function evaluations" <- w162
          "error out" <- w157
          "Waveform Graph 3" <- w145
        }
        frame True {
          w231 = 0.0
          n65 = Build Array(w231, w231, w231, w231) -> (w232:dbl[])
          n66 = Build Array(w231, w233, w231, w231) -> (w234:dbl[])
        }
      }
      "page" <- w92
    }
    "slice" <- w83
  }
  "loss function" <- w40
  "x cut correct 3" <- w19
  "opt param for feedback" <- w18
  n67 = case shown="True" "fit results" {
    tunnel: w15 -> [_ w277]
    tunnel: w14 -> [_ w273]
    tunnel: w13 -> [_ w272]
    tunnel: w12 -> [_ w271]
    tunnel: [w243 w257] -> w11
    tunnel: w10 -> [w243 _]
    tunnel: w1 -> [w242 w256]
    tunnel: w8 -> [w241 w255]
    tunnel: w7 -> [w240 w254]
    tunnel: w6 -> [w239 w253]
    tunnel: [w238 w249] -> w5
    tunnel: [w237 w248] -> w4
    tunnel: [w236 w247] -> w3
    tunnel: [w235 w246] -> w2
    frame False {
      n68 = Build Array(w241) -> (w237:dbl[][])
      n69 = Build Array(w242) -> (w238:dbl[][])
      n70 = Build Array(w240) -> (w236:dbl[][])
      n71 = Build Array(w239) -> (w235:dbl[][])
    }
    frame True {
      n72 = Transpose 2D Array(2D array=w277) -> (transposed array=w276:dbl[][])
      n73 = Transpose 2D Array(2D array=w273) -> (transposed array=w268:dbl[][])
      n74 = Transpose 2D Array(2D array=w272) -> (transposed array=w269:dbl[][])
      n75 = Transpose 2D Array(2D array=w271) -> (transposed array=w270:dbl[][])
      n76 = for {
        tunnel: w276 -> [w313] mode=indexing
        tunnel: [w312] -> w275 mode=indexing
        tunnel: [w311] -> w274 mode=indexing
        tunnel: w270 -> [w300] mode=indexing
        tunnel: w269 -> [w299] mode=indexing
        tunnel: w268 -> [w298] mode=indexing
        tunnel: [w297] -> w267 mode=indexing
        tunnel: [w296] -> w266 mode=indexing
        tunnel: [w295] -> w265 mode=indexing
        tunnel: [w294] -> w264 mode=indexing
        tunnel: [w293] -> w263 mode=indexing
        tunnel: [w292] -> w262 mode=indexing
        tunnel: [w288] -> w244 mode=indexing
        w302 = T7 0 items=["SVD", "Givens", "Givens2", "Householder", "LU Decomposition", "Cholesky", "SVD for Rank Deficient H"] ("algorithm")
        w303 = T8 0 items=["Least Square", "Least Absolute Residual", "Bisquare"] ("method")
        w307 = T7 0 items=["SVD", "Givens", "Givens2", "Householder", "LU Decomposition", "Cholesky", "SVD for Rank Deficient H"] ("algorithm")
        w306 = T8 0 items=["Least Square", "Least Absolute Residual", "Bisquare"] ("method")
        w308 = T7 0 items=["SVD", "Givens", "Givens2", "Householder", "LU Decomposition", "Cholesky", "SVD for Rank Deficient H"] ("algorithm")
        w309 = T8 0 items=["Least Square", "Least Absolute Residual", "Bisquare"] ("method")
        w316 = T7 0 items=["SVD", "Givens", "Givens2", "Householder", "LU Decomposition", "Cholesky", "SVD for Rank Deficient H"] ("algorithm")
        w315 = T8 0 items=["Least Square", "Least Absolute Residual", "Bisquare"] ("method")
        n77 = for {
          N -> [w317]
          tunnel: w313 -> [_] mode=indexing
          tunnel: [w318] -> w301 mode=indexing
          tunnel: [w317] -> w289
          i -> [w318]
        }
        n78 = call <vilib>:"General Polynomial Fit.vi"("Y"=w298, "polynomial order"=4, "X"=w301, "method"=w309, "algorithm"=w308) -> ("Best Polynomial Fit"=w292:dbl[])  [unwired: 7 in, 3 out]
        n79 = call <vilib>:"General Polynomial Fit.vi"("Y"=w300, "polynomial order"=4, "X"=w301, "method"=w303, "algorithm"=w302) -> ("Best Polynomial Fit"=w293:dbl[])  [unwired: 7 in, 3 out]
        n80 = call <vilib>:"General Polynomial Fit.vi"("Y"=w313, "polynomial order"=4, "X"=w301, "method"=w315, "algorithm"=w316) -> ("Best Polynomial Fit"=w311:dbl[])  [unwired: 7 in, 3 out]
        n81 = call <vilib>:"General Polynomial Fit.vi"("Y"=w299, "polynomial order"=1, "X"=w301, "method"=w306, "algorithm"=w307) -> ("Best Polynomial Fit"=w294:dbl[], "Polynomial Coefficients"=w291:dbl[])  [unwired: 7 in, 2 out]
        n82 = Subtract(x=w293, y=w300) -> (x-y=w297:dbl[])
        n83 = Subtract(x=w311, y=w313) -> (x-y=w312:dbl[])
        n84 = Subtract(x=w294, y=w299) -> (x-y=w296:dbl[])
        n85 = Subtract(x=w292, y=w298) -> (x-y=w295:dbl[])
        n86 = Index Array(array=w291) -> (element #2=w290:dbl)  [unwired: 2 in, 1 out]
        n87 = Multiply(x=w290, y=w289) -> (x*y=w288:dbl)
      }
      "x cut pos fit" <- w265
      "r correct fit" <- w275
      "y correct fit" <- w266
      "intensity correct fit" <- w267
      "y correct" <- w244
      n88 = Transpose 2D Array(2D array=w262) -> (transposed array=w260:dbl[][])
      n89 = Transpose 2D Array(2D array=w264) -> (transposed array=w259:dbl[][])
      n90 = Transpose 2D Array(2D array=w274) -> (transposed array=w261:dbl[][])
      n91 = Transpose 2D Array(2D array=w263) -> (transposed array=w258:dbl[][])
      n92 = for {
        tunnel: w261 -> [w281] mode=indexing
        tunnel: w260 -> [w280] mode=indexing
        tunnel: w259 -> [w279] mode=indexing
        tunnel: w258 -> [w278] mode=indexing
        tunnel: [w282] -> w257 mode=indexing
        tunnel: [w281] -> w252 mode=concatenating
        tunnel: [w280] -> w251 mode=concatenating
        tunnel: [w279] -> w250 mode=concatenating
        tunnel: [w278] -> w245 mode=concatenating
        n93 = for {
          tunnel: w281 -> [w287] mode=indexing
          tunnel: w280 -> [w286] mode=indexing
          tunnel: w279 -> [w285] mode=indexing
          tunnel: w278 -> [w284] mode=indexing
          tunnel: [w283] -> w282 mode=indexing
          n94 = Build Array(w287, w286, w285, w284) -> (w283:dbl[])
        }
      }
      n95 = Build Array(w256, w252) -> (w249:dbl[][])
      n96 = Build Array(w255, w251) -> (w248:dbl[][])
      n97 = Build Array(w254, w250) -> (w247:dbl[][])
      n98 = Build Array(w253, w245) -> (w246:dbl[][])
    }
  }
  "r correct" <- w5
  "x cut pos" <- w4
  "y correct" <- w3
  "intensity correct" <- w2
  "optimized parameters" <- w11
  n99 = Add(x=w28, y=w1) -> (x+y=w26:dbl[])
  n100 = Divide(x=w27, y=w28) -> (x/y=w25:dbl)
  n101 = Divide(x=w27, y=w26) -> (x/y=w24:dbl[])
  n102 = Subtract(x=w25, y=w24) -> (x-y=w23:dbl[])
  n103 = Divide(x=w23, y=2.0) -> (x/y=w22:dbl[])
  n104 = Subtract(x=w19, y=w22) -> (x-y=→"x cut correct 2":dbl[])
